vi "Main.vi"() -> ()   [LabVIEW 2018] (continued)
              n599 = Greater Or Equal?(x=w1197, y=w1212) -> (x >= y?=w1196:bool)
              n600 = Divide(x=w1197, y=w1212) -> (x/y=w1209:dbl)
              n601 = Compound Arithmetic op=OR(w1220, "Stop Measure", w1196) -> (w1219:bool)
              n602 = Reshape Array(w1200, w1199, w1199) -> (w1201:dbl[][])
              n603 = Reshape Array(w1202, w1199, w1199) -> (w1203:dbl[][])
              n604 = Reshape Array(w1204, w1199, w1199) -> (w1205:dbl[][])
              n605 = Reshape Array(w1207, w1199, w1199) -> (w1206:dbl[][])
              n606 = Reshape Array(w1218, w1199, w1199) -> (w1208:dbl[][])
              n607 = Multiply(x=w1209, y=100.0) -> (x*y=→"Meas Progress":dbl)
              n608 = local read "V_IF (0.5pi)"() -> (w1214:dbl[][])
              n609 = local read "V_IF (1.5pi)"() -> (w1216:dbl[][])
              n610 = local read "V_IF (pi)"() -> (w1215:dbl[][])
              n611 = local read "V_IF (0)"() -> (w1213:dbl[][])
              n612 = local read "V_DC"() -> (w1217:dbl[][])
              n613 = local read "Shutter Line"() -> (w1177:tag)
              n614 = call "RunningAverage.vi"("New Image"=w1206, "# of Averages for the Old Image"=w1198, "Old Image"=w1216) -> ("Averaged Image"=w1179:dbl[][])  [unwired: 8 in]
              "V_IF (1.5pi)" <- w1179
              n615 = call "RunningAverage.vi"("New Image"=w1201, "# of Averages for the Old Image"=w1198, "Old Image"=w1213) -> ("Averaged Image"=w1182:dbl[][])  [unwired: 8 in]
              "V_IF (0)" <- w1182
              n616 = call "RunningAverage.vi"("New Image"=w1203, "# of Averages for the Old Image"=w1198, "Old Image"=w1214) -> ("Averaged Image"=w1181:dbl[][])  [unwired: 8 in]
              "V_IF (0.5pi)" <- w1181
              n617 = call "RunningAverage.vi"("New Image"=w1205, "# of Averages for the Old Image"=w1198, "Old Image"=w1215) -> ("Averaged Image"=w1180:dbl[][])  [unwired: 8 in]
              "V_IF (pi)" <- w1180
              n618 = call "RunningAverage.vi"("New Image"=w1208, "# of Averages for the Old Image"=w1198, "Old Image"=w1217) -> ("Averaged Image"=w1178:dbl[][])  [unwired: 8 in]
              "V_DC" <- w1178
              n619 = call "ShutterControl.vi"("error in"=w1186, "Shutter Line"=w1177, "Shutter"=FALSE) -> ("error out"=w1188:errorcluster, "Status Indicator"=w1190:bool)  [unwired: 7 in]
              n620 = local write "Shutter"(w1190) -> ()
            }
            n621 = local read "[d13]"() -> (w1141:dbl)
            n622 = local read "[d24]"() -> (w1140:dbl)
            n623 = call "DAQClose.vi"("error in"=w1166, "Functions"=w1167, "Tasks In"=w1168, "DAQ Channels"=w1169) -> ("error out"=w1152:errorcluster)  [unwired: 7 in]
            n624 = local read "[M/B]"() -> (w1145:dbl)
            n625 = local read "[O_B]"() -> (w1144:dbl)
            n626 = call "GSCalculation.vi"("[d24]"=w1140, "[d13]"=w1141, "[O_B]"=w1144, "V_DC"=w1146, "[M/B]"=w1145, "V_IF (1.5pi)"=w1148, "V_IF (pi)"=w1149, "V_IF (0.5pi)"=w1150, "V_IF (0)"=w1151) -> ("S"=w1142:dbl[][], "G"=w1143:dbl[][])  [unwired: 1 in]
            "G Data" <- w1143
            "S Data" <- w1142
          }
          frame #2 {
            n627 = case shown="True" "Calculate Lifetimes and Phasors During Image Acquisition?" {
              tunnel: w1239 -> [w1242 w1272]
              tunnel: w1238 -> [_ w1264]
              tunnel: w1237 -> [_ w1251]
              tunnel: w1236 -> [_ w1250]
              tunnel: w1235 -> [_ w1249]
              tunnel: [w1242 w1244] -> w1234
              frame False {
                # "If need to be fast, e.g., 3D stack acquisition"
              }
              frame True {
                # "If do lifetime and other calcuations"
                n628 = Square(x=w1264) -> (x^2=w1282:i32)
                n629 = call "LifetimeCalculation.vi"("LaserRepRate"="LaserRepRate (Hz)", "S"=w1249, "G"=w1250) -> ("DC&1w Lifetime"=w1273:dbl[][], "1w Lifetime"=w1274:dbl[][])  [unwired: 7 in]
                "1w Lifetime (s)" <- w1274
                "DC&1w Lifetime (s)" <- w1273
                n630 = control-ref of="1w Lifetime Hist"() -> (w1284:refnum<vi>)
                n631 = control-ref of="DC&1w Lifetime Hist"() -> (w1283:refnum<vi>)
                n632 = control-ref of="Lifetime Color Ramp"() -> (w1266:refnum<vi>)
                n633 = control-ref of="Phasor Plot"() -> (w1258:refnum<vi>)
                n634 = local read "Auto Scale?"() -> (w1246:bool)
                n635 = control-ref of="Composite Image"() -> (w1267:refnum<vi>)
                n636 = control-ref of="Image with Phasors"() -> (w1261:refnum<vi>)
                n637 = call "LifetimeHistogram.vi"("1w Lifetime"=w1274, "DC&1w Lifetime"=w1273, "1w reference"=w1284, "DC&1w reference"=w1283, "Max Lifetime (s)"="Max Lifetime (s)", "Min Lifetime (s)"="Min Lifetime (s)", "Data Size"=w1282, "error in (no error)"=w1272, "Bins"="Bins") -> ("error out"=w1268:errorcluster, "1w Lifetime Hist"=→"1w Lifetime Hist":T7, "DC&1w Lifetime Hist"=→"DC&1w Lifetime Hist":T7, "1w mean"=→"u_1w":dbl, "1w std"=→"std_1":dbl, "DC&1w mean"=→"u_01":dbl, "DC&1w std"=→"std_01":dbl)  [unwired: 4 in]
                n638 = case shown="\"1w Lifetime\", Default" "Lifetime Selection" {
                  tunnel: w1274 -> [w1288 _]
                  tunnel: w1273 -> [_ w1289]
                  tunnel: [w1288 w1289] -> w1271
                  frame "1w Lifetime", Default {
                  }
                  frame "DC&1w Lifetime" {
                  }
                }
                n639 = call "HSVCombIntensityLifetime.vi"("min_intensity"="Min Intensity", "Auto Scale?"=w1246, "max_intensity"="Max Intensity", "lifetime_max (s)"="Max Lifetime (s)", "lifetime_min (s)"="Min Lifetime (s)", "Lifetime image"=w1271, "Intensity image"=w1251) -> ("Min"=w1247:dbl, "Max"=w1248:dbl, "Lifetime Color Ramp"=→"Lifetime Color Ramp":i32[][], "HSV to RGB Picture"=→"Composite Image":picture)  [unwired: 1 in]
                n640 = call "Array2GrayPic.vi"("Pic Reference"=w1261, "Threshold (min)"=w1247, "Threshold (max)"=w1248, "Auto Scale?"=w1246, "Intensity"=w1251) -> ("Gray Picture"=→"Image with Phasors":picture)  [unwired: 6 in]
                n641 = local write "Max Intensity"(w1248) -> ()
                n642 = local write "Min Intensity"(w1247) -> ()
                n643 = property on="V_DC" class="IntGraph (strict)"(error in=w1268, "ZScale.Maximum"=w1248, "ZScale.Minimum"=w1247) -> (error out=w1265:errorcluster)  [unwired: 1 in, 1 out]
                n644 = call "CompositeProperties.vi"("Image Reference"=w1267, "Ramp Reference"=w1266, "Pixel Size"=w1264, "Max Lifetime (s)"="Max Lifetime (s)", "Min Lifetime (s)"="Min Lifetime (s)", "error in (no error)"=w1265) -> ("error out"=w1245:errorcluster)  [unwired: 13 in]
                n645 = call "DrawPhasorPlot.vi"("Intensity"=w1251, "G Data"=w1250, "S Data"=w1249, "Threshold (max)"=w1248, "Threshold (min)"=w1247, "error in"=w1245, "G_max"="G_max", "Auto Scale?"=w1246, "G_min"="G_min", "Phasor Grids"="Phasor Grids", "S_max"="S_max", "Reference"=w1258, "S_min"="S_min", "Phasor Colormap"="Phasor Colormap") -> ("Phasor Plot"=→"Phasor Plot":dbl[][], "error out"=w1244:errorcluster)  [unwired: 4 in]
              }
            }
          }
          frame #3 {
            w1297 = FALSE ("Fast Scan")
            n646 = Tick Count (ms)() -> (millisecond timer value=w1293:u32)
            n647 = local write "Measure"(w1297) -> ()
            n648 = local write "Stop Measure"(w1297) -> ()
            n649 = Subtract(x=w1293, y=w1292) -> (x-y=w1294:u32)
            n650 = To Double Precision Float(number=w1294) -> (double precision float=w1295:dbl)
            n651 = Divide(x=w1295, y=1000.0) -> (x/y=→"Actual Meas Time (s)":dbl)
          }
        }
      }
      event "Refresh": Value Change {
        n652 = event-data() -> ()  [unwired: 1 in, 1 out]
        n653 = flat-sequence {
          tunnel: [w1348] -> w1306
          tunnel: w1305 -> [w1348]
          tunnel: [w1346] -> w1303
          tunnel: w1302 -> [w1347]
          tunnel: w1306 -> [w1359]
          tunnel: [w1359] -> w1304
          tunnel: w1303 -> [w1358]
          tunnel: [w1358] -> w1301
          frame #0 {
            n654 = local read "Measurement Parameters"() -> (w1350:T4)
            n655 = local read "LaserRepRate (Hz)"() -> (w1307:dbl)
            n656 = Unbundle By Name(w1350) -> ("Pixel Size"=w1349:dbl)
            n657 = local read "G Data"() -> (w1352:dbl[][])
            n658 = local read "V_DC"() -> (w1354:dbl[][])
            n659 = local read "S Data"() -> (w1353:dbl[][])
            n660 = To Long Integer(number=w1349) -> (32bit integer=w1351:i32)
            n661 = Square(x=w1351) -> (x^2=w1345:i32)
            n662 = local read "Phasor Colormap"() -> (w1310:T8)
            n663 = local read "Max Lifetime (s)"() -> (w1339:dbl)
            n664 = local read "Min Lifetime (s)"() -> (w1338:dbl)
            n665 = control-ref of="Phasor Plot"() -> (w1309:refnum<vi>)
            n666 = control-ref of="Lifetime Color Ramp"() -> (w1319:refnum<vi>)
            n667 = call "LifetimeCalculation.vi"("LaserRepRate"=w1307, "S"=w1353, "G"=w1352) -> ("DC&1w Lifetime"=w1334:dbl[][], "1w Lifetime"=w1335:dbl[][])  [unwired: 7 in]
            n668 = local read "Bins"() -> (w1333:i32)
            n669 = control-ref of="1w Lifetime Hist"() -> (w1326:refnum<vi>)
            n670 = control-ref of="DC&1w Lifetime Hist"() -> (w1325:refnum<vi>)
            n671 = local read "Phasor Grids"() -> (w1311:i32)
            n672 = local read "Max Intensity"() -> (w1337:dbl)
            n673 = local read "Min Intensity"() -> (w1336:dbl)
            n674 = local read "Auto Scale?"() -> (w1341:bool)
            n675 = local read "G_max"() -> (w1315:dbl)
            n676 = local read "S_max"() -> (w1313:dbl)
            n677 = local read "G_min"() -> (w1314:dbl)
            n678 = local read "S_min"() -> (w1312:dbl)
            n679 = control-ref of="Image with Phasors"() -> (w1318:refnum<vi>)
            n680 = control-ref of="Composite Image"() -> (w1320:refnum<vi>)
            n681 = call "LifetimeHistogram.vi"("1w Lifetime"=w1335, "DC&1w Lifetime"=w1334, "1w reference"=w1326, "DC&1w reference"=w1325, "Max Lifetime (s)"=w1339, "Min Lifetime (s)"=w1338, "Data Size"=w1345, "error in (no error)"=w1347, "Bins"=w1333) -> ("error out"=w1343:errorcluster, "1w Lifetime Hist"=w1332:T7, "DC&1w Lifetime Hist"=w1331:T7, "1w mean"=w1330:dbl, "1w std"=w1329:dbl, "DC&1w mean"=w1328:dbl, "DC&1w std"=w1327:dbl)  [unwired: 4 in]
            n682 = local write "1w Lifetime (s)"(w1335) -> ()
            n683 = local write "DC&1w Lifetime (s)"(w1334) -> ()
            n684 = local write "1w Lifetime Hist"(w1332) -> ()
            n685 = local write "DC&1w Lifetime Hist"(w1331) -> ()
            n686 = local write "u_1w"(w1330) -> ()
            n687 = local write "std_1"(w1329) -> ()
            n688 = local write "u_01"(w1328) -> ()
            n689 = local write "std_01"(w1327) -> ()
            n690 = local read "Lifetime Selection"() -> (w1308:enum32{"1w Lifetime", "DC&1w Lifetime"})
            n691 = case shown="\"1w Lifetime\", Default" w1308 {
              tunnel: w1335 -> [w1355 _]
              tunnel: w1334 -> [_ w1356]
              tunnel: [w1355 w1356] -> w1344
              frame "1w Lifetime", Default {
              }
              frame "DC&1w Lifetime" {
              }
            }
            n692 = call "HSVCombIntensityLifetime.vi"("min_intensity"=w1336, "Auto Scale?"=w1341, "max_intensity"=w1337, "lifetime_max (s)"=w1339, "lifetime_min (s)"=w1338, "Lifetime image"=w1344, "Intensity image"=w1354) -> ("Min"=w1321:dbl, "Max"=w1322:dbl, "Lifetime Color Ramp"=w1323:i32[][], "HSV to RGB Picture"=w1324:picture)  [unwired: 1 in]
            n693 = call "Array2GrayPic.vi"("Pic Reference"=w1318, "Threshold (min)"=w1321, "Threshold (max)"=w1322, "Auto Scale?"=w1341, "Intensity"=w1354) -> ("Gray Picture"=w1317:picture)  [unwired: 6 in]
            n694 = local write "Image with Phasors"(w1317) -> ()
            n695 = property on="V_DC" class="IntGraph (strict)"(error in=w1343, "ZScale.Maximum"=w1322, "ZScale.Minimum"=w1321) -> (error out=w1342:errorcluster)  [unwired: 1 in, 1 out]
            n696 = call "CompositeProperties.vi"("Image Reference"=w1320, "Ramp Reference"=w1319, "Pixel Size"=w1351, "Max Lifetime (s)"=w1339, "Min Lifetime (s)"=w1338, "error in (no error)"=w1342) -> ("error out"=w1340:errorcluster)  [unwired: 13 in]
            n697 = call "DrawPhasorPlot.vi"("Intensity"=w1354, "G Data"=w1352, "S Data"=w1353, "Threshold (max)"=w1322, "Threshold (min)"=w1321, "error in"=w1340, "G_max"=w1315, "Auto Scale?"=w1341, "G_min"=w1314, "Phasor Grids"=w1311, "S_max"=w1313, "Reference"=w1309, "S_min"=w1312, "Phasor Colormap"=w1310) -> ("Phasor Plot"=w1316:dbl[][], "error out"=w1346:errorcluster)  [unwired: 4 in]
            n698 = local write "Phasor Plot"(w1316) -> ()
            n699 = local write "Composite Image"(w1324) -> ()
            n700 = local write "Lifetime Color Ramp"(w1323) -> ()
            n701 = local write "Max Intensity"(w1322) -> ()
            n702 = local write "Min Intensity"(w1321) -> ()
          }
          frame #1 {
            n703 = local write "Refresh"(FALSE ("Fast Scan")) -> ()
          }
        }
      }
      event "Z-Stack Measure": Value Change {
        n704 = event-data() -> ()  [unwired: 1 in, 1 out]
        n705 = local read "Current Slice"() -> (w1370:i32)
        n706 = Divide(x=w1370, y="Z Slice Number") -> (x/y=w1378:dbl)
        n707 = Greater Or Equal?(x=w1370, y="Z Slice Number") -> (x >= y?=w1371:bool)
        n708 = Multiply(x=w1378, y=100.0) -> (x*y=→"Stack Progress":dbl)
        n709 = local read "Use Stage?"() -> (w1360:bool)
        n710 = Equal To 0?(x=w1370) -> (x = 0?=w1369:bool)
        n711 = case shown="True" w1369 {
          tunnel: w1380 -> [w1440 w1473]
          tunnel: w1381 -> [w1439 w1474]
          tunnel: [w1438 w1472] -> w1374
          tunnel: [w1437 w1471] -> w1372
          tunnel: w1371 -> [w1433 _]
          tunnel: [FALSE ("Stop Stack Measure") w1468] -> w1362
          tunnel: w1360 -> [w1425 w1466]
          frame False {
            # "Continue measurement , move stage"
            n712 = case shown="False" w1433 {
              tunnel: w1440 -> [w1445 w1464]
              tunnel: w1439 -> [w1444 w1465]
              tunnel: [w1443 w1465] -> w1438
              tunnel: [w1442 w1464] -> w1437
              tunnel: w1425 -> [w1441 _]
              frame False {
                n713 = case shown="True" w1441 {
                  tunnel: w1445 -> [w1446 w1463]
                  tunnel: w1444 -> [w1447 w1462]
                  tunnel: [w1447 w1450] -> w1443
                  tunnel: [w1446 w1448] -> w1442
                  frame False {
                  }
                  frame True {
                    # "Moves up by 1 step defined by \nthe 'C' command"
                    n714 = Number To Decimal String(number="Z Slice Size (.1um)") -> (decimal integer string=w1456:string)  [unwired: 1 in]
                    n715 = Concatenate Strings("C" ("string"), "," ("string"), w1456, "\r", "U" ("string")) -> (w1453:string)
                    n716 = VISA Write(VISA resource name=w1462, write buffer=w1453, error in (no error)=w1463) -> (VISA resource name out=w1460:refnum<visa-resource-name>, error out=w1459:errorcluster)  [unwired: 1 out]
                    n717 = VISA Read(VISA resource name=w1460, byte count=u32 256, error in (no error)=w1459) -> (VISA resource name out=w1451:refnum<visa-resource-name>, error out=w1449:errorcluster)  [unwired: 2 out]
                    n718 = VISA Clear(VISA resource name=w1451, error in (no error)=w1449) -> (VISA resource name out=w1450:refnum<visa-resource-name>, error out=w1448:errorcluster)
                  }
                }
              }
              frame True {
              }
            }
            n719 = local read "3D Intensity"() -> (w1434:dbl[][][])
            n720 = local read "G Data"() -> (w1432:dbl[][])
            n721 = local read "S Data"() -> (w1431:dbl[][])
            n722 = local read "V_DC"() -> (w1436:dbl[][])
            n723 = local read "3D G"() -> (w1428:dbl[][][])
            n724 = local read "3D S"() -> (w1427:dbl[][][])
            n725 = Build Array (concatenate)(w1434, w1436) -> (→"3D Intensity":dbl[][][])
            n726 = Build Array (concatenate)(w1428, w1432) -> (→"3D G":dbl[][][])
            n727 = Build Array (concatenate)(w1427, w1431) -> (→"3D S":dbl[][][])
          }
          frame True {
            # "Beginning the measurment, record current Z position"
            n728 = local read "3D Time-Lapse Measure"() -> (w1467:bool)
            n729 = case shown="False" w1467 {
              tunnel: [w1487 TRUE ("T button?")] -> w1469
              frame False {
                n730 = Two Button Dialog(message="Discard Previous Stack?") -> (T button?=w1487:bool)  [unwired: 2 in]
              }
              frame True {
              }
            }
            n731 = case shown="True" w1466 {
              tunnel: w1474 -> [w1476 w1482]
              tunnel: w1473 -> [w1475 w1481]
              tunnel: [w1476 w1480] -> w1472
              tunnel: [w1475 w1479] -> w1471
              frame False {
              }
              frame True {
                n732 = VISA Write(VISA resource name=w1482, write buffer="PZ" ("string"), error in (no error)=w1481) -> (VISA resource name out=w1484:refnum<visa-resource-name>, error out=w1485:errorcluster)  [unwired: 1 out]
                n733 = VISA Read(VISA resource name=w1484, byte count=u32 256, error in (no error)=w1485) -> (VISA resource name out=w1480:refnum<visa-resource-name>, read buffer=w1478:string, error out=w1479:errorcluster)  [unwired: 1 out]
                n734 = Decimal String To Number(string=w1478) -> (number=→"Initial Z Pos (.1um)":i32)  [unwired: 2 in, 1 out]
              }
            }
            n735 = local write "Calculate Lifetimes and Phasors During Image Acquisition?"(FALSE ("Calculate Lifetimes and Phasors During Image Acquisition?")) -> ()
            n736 = case shown="True" w1469 {
              tunnel: [TRUE ("Stop Stack Measure") FALSE ("Stop Stack Measure")] -> w1468
              frame False {
              }
              frame True {
                w1492 = dbl[][][] [] ("3D Intensity (BT)")
                n737 = local write "3D Intensity"(w1492) -> ()
                n738 = local write "3D G"(w1492) -> ()
                n739 = local write "3D S"(w1492) -> ()
              }
            }
          }
        }
        n740 = Compound Arithmetic op=OR(w1371, "Stop Stack Measure", w1362) -> (w1375:bool)
        n741 = case shown="True" w1375 {
          tunnel: w1374 -> [w1394 w1399]
          tunnel: w1372 -> [w1389 w1398]
          tunnel: [w1394 w1404] -> w1368
          tunnel: [w1391 w1400] -> w1366
          tunnel: w1370 -> [w1393 _]
          frame False {
            n742 = Increment(x=w1393) -> (x+1=→"Current Slice":i32)
            n743 = property on="Measure" class="Bool (strict)"(error in=w1389, "Val(Sgnl)"=TRUE ("Value (Signaling)")) -> (error out=w1388:errorcluster)  [unwired: 1 in, 1 out]
            n744 = property on="Z-Stack Measure" class="Bool (strict)"(error in=w1388, "Val(Sgnl)"=TRUE ("Value (Signaling)")) -> (error out=w1391:errorcluster)  [unwired: 1 in, 1 out]
          }
          frame True {
            w1403 = FALSE ("Fast Scan")
            n745 = local read "Use Stage?"() -> (w1396:bool)
            n746 = case shown="True" w1396 {
              tunnel: [w1407 w1411] -> w1404
              tunnel: [w1406 w1410] -> w1401
              tunnel: w1399 -> [w1407 w1409]
              tunnel: w1398 -> [w1406 w1408]
              frame False {
              }
              frame True {
                n747 = local read "Initial Z Pos (.1um)"() -> (w1419:i32)
                n748 = Number To Decimal String(number=w1419) -> (decimal integer string=w1416:string)  [unwired: 1 in]
                n749 = Concatenate Strings("GZ" ("string"), "," ("string"), w1416) -> (w1418:string)
                n750 = VISA Write(VISA resource name=w1409, write buffer=w1418, error in (no error)=w1408) -> (VISA resource name out=w1413:refnum<visa-resource-name>, error out=w1414:errorcluster)  [unwired: 1 out]
                n751 = VISA Read(VISA resource name=w1413, byte count=u32 256, error in (no error)=w1414) -> (VISA resource name out=w1411:refnum<visa-resource-name>, error out=w1410:errorcluster)  [unwired: 2 out]
              }
            }
            n752 = local read "3D Time-Lapse Measure"() -> (w1402:bool)
            n753 = local write "Calculate Lifetimes and Phasors During Image Acquisition?"(TRUE ("Calculate Lifetimes and Phasors During Image Acquisition?")) -> ()
            n754 = local write "Stop Stack Measure"(w1403) -> ()
            n755 = local write "Z-Stack Measure"(w1403) -> ()
            n756 = local write "Current Slice"(0 ("Current Slice")) -> ()
            n757 = case shown="True" w1402 {
              tunnel: w1401 -> [w1420 w1422]
              tunnel: [w1420 w1421] -> w1400
              frame False {
              }
              frame True {
                w1423 = TRUE ("Value (Signaling)")
                n758 = property on="Save 3D Stacks" class="Bool (strict)"(error in=w1422, "Val(Sgnl)"=w1423) -> (error out=w1424:errorcluster)  [unwired: 1 in, 1 out]
                n759 = property on="3D Time-Lapse Measure" class="Bool (strict)"(error in=w1424, "Val(Sgnl)"=w1423) -> (error out=w1421:errorcluster)  [unwired: 1 in, 1 out]
              }
            }
          }
        }
        n760 = local read "Use Stage?"() -> (w1361:bool)
        n761 = case shown="False" w1361 {
          tunnel: w1368 -> [w1382 w1387]
          tunnel: [w1382 w1386] -> w1367
          tunnel: w1366 -> [w1383 w1385]
          tunnel: [w1383 w1384] -> w1365
          frame False {
          }
          frame True {
            n762 = VISA Clear(VISA resource name=w1387, error in (no error)=w1385) -> (VISA resource name out=w1386:refnum<visa-resource-name>, error out=w1384:errorcluster)
          }
        }
      }
      event "3D Stack to Show", "Slice Slider": Value Change {
        n763 = event-data() -> ()  [unwired: 1 in, 1 out]
        n764 = local read "3D Intensity"() -> (w1515:dbl[][][])
        n765 = local read "Max Lifetime (s)"() -> (w1517:dbl)
        n766 = local read "Min Lifetime (s)"() -> (w1516:dbl)
        n767 = local read "LaserRepRate (Hz)"() -> (w1493:dbl)
        n768 = case shown="False" "Auto Scale?" {
          tunnel: w1515 -> [_ w1535]
          tunnel: [w1532 w1534] -> w1514
          tunnel: [w1531 w1533] -> w1513
          frame False {
            n769 = local read "Max Intensity"() -> (w1532:dbl)
            n770 = local read "Min Intensity"() -> (w1531:dbl)
          }
          frame True {
            n771 = Array Max & Min(array=w1535) -> (max value=w1534:dbl, min value=w1533:dbl)  [unwired: 2 out]
          }
        }
        n772 = local read "3D G"() -> (w1499:dbl[][][])
        n773 = local read "3D S"() -> (w1498:dbl[][][])
        n774 = control-ref of="Slice of 3D Stack"() -> (w1500:refnum<vi>)
        n775 = Multiply(x=w1493, y=6.283185307179586) -> (x*y=w1496:dbl)
        n776 = case shown="\"Overlap 3D\"" "3D Stack to Show" {
          tunnel: "Slice Slider" -> [w1545 w1558 w1574 w1591 w1612 w1632 w1651]
          tunnel: [w1543 w1557 w1573 w1592 w1611 w1635 w1654] -> w1518
          tunnel: w1517 -> [_ w1553 w1570 w1584 w1602 _ _]
          tunnel: w1516 -> [_ w1552 w1569 w1583 w1595 _ _]
          tunnel: w1515 -> [w1542 _ _ w1590 w1610 w1636 w1655]
          tunnel: w1514 -> [w1538 _ _ w1587 w1605 w1621 w1646]
          tunnel: w1513 -> [w1537 _ _ w1586 w1604 w1620 w1645]
          tunnel: [w1536 w1551 w1568 w1581 w1607 w1616 w1648] -> w1502
          tunnel: w1500 -> [w1540 w1555 w1567 w1589 w1608 w1617 w1650]
          tunnel: w1499 -> [_ w1549 w1564 w1579 w1597 w1634 w1653]
          tunnel: w1498 -> [_ w1548 _ w1578 _ w1633 w1652]
          tunnel: w1496 -> [_ w1547 w1561 w1577 w1596 _ _]
          frame "Intensity 3D", Default {
            n777 = Array Size(array=w1542) -> (size(s)=w1544:i32[])
            n778 = Index Array(array=w1542, index (dim 0)=w1545) -> (element=w1541:dbl[][])  [unwired: 2 in]
            n779 = Index Array(array=w1544) -> (element=w1543:i32)  [unwired: 1 in]
            n780 = call "Array2GrayPic.vi"("Pic Reference"=w1540, "Threshold (min)"=w1537, "Threshold (max)"=w1538, "Auto Scale?"=FALSE, "Intensity"=w1541) -> ("Gray Picture"=w1536:picture)  [unwired: 6 in]
          }
          frame "1w Lifetime 3D" {
            n781 = Divide(x=w1548, y=w1549) -> (x/y=w1550:dbl[][][])
            n782 = Divide(x=w1550, y=w1547) -> (x/y=w1546:dbl[][][])
            n783 = Array Size(array=w1546) -> (size(s)=w1559:i32[])
            n784 = Index Array(array=w1546, index (dim 0)=w1558) -> (element=w1554:dbl[][])  [unwired: 2 in]
            n785 = Index Array(array=w1559) -> (element=w1557:i32)  [unwired: 1 in]
            n786 = call "Array2GrayPic.vi"("Pic Reference"=w1555, "Threshold (min)"=w1552, "Threshold (max)"=w1553, "Auto Scale?"=FALSE, "Intensity"=w1554) -> ("Gray Picture"=w1551:picture)  [unwired: 6 in]
          }
          frame "DC&1w Lifetime 3D" {
            n787 = Divide(x=1.0, y=w1564) -> (x/y=w1563:dbl[][][])
            n788 = Decrement(x=w1563) -> (x-1=w1566:dbl[][][])
            n789 = Square Root(x=w1566) -> (sqrt(x)=w1562:dbl[][][])
            n790 = Divide(x=w1562, y=w1561) -> (x/y=w1560:dbl[][][])
            n791 = Array Size(array=w1560) -> (size(s)=w1575:i32[])
            n792 = Index Array(array=w1560, index (dim 0)=w1574) -> (element=w1571:dbl[][])  [unwired: 2 in]
            n793 = Index Array(array=w1575) -> (element=w1573:i32)  [unwired: 1 in]
            n794 = call "Array2GrayPic.vi"("Pic Reference"=w1567, "Threshold (min)"=w1569, "Threshold (max)"=w1570, "Auto Scale?"=FALSE, "Intensity"=w1571) -> ("Gray Picture"=w1568:picture)  [unwired: 6 in]
          }
          frame "1w Composite 3D" {
            n795 = Divide(x=w1578, y=w1579) -> (x/y=w1580:dbl[][][])
            n796 = Divide(x=w1580, y=w1577) -> (x/y=w1576:dbl[][][])
            n797 = Index Array(array=w1576, index (dim 0)=w1591) -> (element=w1585:dbl[][])  [unwired: 2 in]
            n798 = Index Array(array=w1590, index (dim 0)=w1591) -> (element=w1588:dbl[][])  [unwired: 2 in]
            n799 = Array Size(array=w1590) -> (size(s)=w1593:i32[])
            n800 = Index Array(array=w1593) -> (element=w1592:i32)  [unwired: 1 in]
            n801 = call "Array2HSVColorPic.vi"("Intensity"=w1588, "Threshold (max)"=w1587, "Threshold (min)"=w1586, "Lifetime"=w1585, "lifetime_max (s)"=w1584, "lifetime_min (s)"=w1583, "Pic Reference"=w1589, "Auto Scale?"=FALSE) -> ("Gray Picture"=w1581:picture)  [unwired: 11 in]
          }
          frame "DC&1w Composite 3D" {
            n802 = Divide(x=1.0, y=w1597) -> (x/y=w1599:dbl[][][])
            n803 = Decrement(x=w1599) -> (x-1=w1601:dbl[][][])
            n804 = Square Root(x=w1601) -> (sqrt(x)=w1598:dbl[][][])
            n805 = Divide(x=w1598, y=w1596) -> (x/y=w1594:dbl[][][])
            n806 = Index Array(array=w1594, index (dim 0)=w1612) -> (element=w1603:dbl[][])  [unwired: 2 in]
            n807 = Index Array(array=w1610, index (dim 0)=w1612) -> (element=w1606:dbl[][])  [unwired: 2 in]
            n808 = Array Size(array=w1610) -> (size(s)=w1613:i32[])
            n809 = Index Array(array=w1613) -> (element=w1611:i32)  [unwired: 1 in]
            n810 = call "Array2HSVColorPic.vi"("Intensity"=w1606, "Threshold (max)"=w1605, "Threshold (min)"=w1604, "Lifetime"=w1603, "lifetime_max (s)"=w1602, "lifetime_min (s)"=w1595, "Pic Reference"=w1608, "Auto Scale?"=FALSE) -> ("Gray Picture"=w1607:picture)  [unwired: 11 in]
          }
          frame "Phasor 3D" {
            # "Transpose"
            n811 = Array Size(array=w1636) -> (size(s)=w1637:i32[])
            n812 = Index Array(array=w1633, index (dim 0)=w1632) -> (element=w1622:dbl[][])  [unwired: 2 in]
            n813 = Index Array(array=w1634, index (dim 0)=w1632) -> (element=w1623:dbl[][])  [unwired: 2 in]
            n814 = Index Array(array=w1636, index (dim 0)=w1632) -> (element=w1624:dbl[][])  [unwired: 2 in]
            n815 = Index Array(array=w1637) -> (element=w1635:i32)  [unwired: 1 in]
            n816 = local read "Phasor Colormap"() -> (w1625:T8)
            n817 = local read "G_max"() -> (w1631:dbl)
            n818 = local read "S_max"() -> (w1629:dbl)
            n819 = local read "G_min"() -> (w1630:dbl)
            n820 = local read "S_min"() -> (w1628:dbl)
            n821 = control-ref of="Phasor Plot"() -> (w1626:refnum<vi>)
            n822 = local read "Phasor Grids"() -> (w1627:i32)
            n823 = call "DrawPhasorPlot.vi"("Intensity"=w1624, "G Data"=w1623, "S Data"=w1622, "Threshold (max)"=w1621, "Threshold (min)"=w1620, "G_max"=w1631, "Auto Scale?"=FALSE, "G_min"=w1630, "Phasor Grids"=w1627, "S_max"=w1629, "Reference"=w1626, "S_min"=w1628, "Phasor Colormap"=w1625) -> ("Phasor Plot"=w1614:dbl[][])  [unwired: 5 in, 1 out]
            n824 = Transpose 2D Array(2D array=w1614) -> (transposed array=w1615:dbl[][])
            n825 = call "Array2GrayPic.vi"("Pic Reference"=w1617, "Auto Scale?"=TRUE, "Intensity"=w1615) -> ("Gray Picture"=w1616:picture)  [unwired: 8 in]
          }
          frame "Overlap 3D" {
            n826 = Array Size(array=w1655) -> (size(s)=w1656:i32[])
            n827 = Index Array(array=w1655, index (dim 0)=w1651) -> (element=w1649:dbl[][])  [unwired: 2 in]
            n828 = Index Array(array=w1652, index (dim 0)=w1651) -> (element=w1643:dbl[][])  [unwired: 2 in]
            n829 = Index Array(array=w1653, index (dim 0)=w1651) -> (element=w1644:dbl[][])  [unwired: 2 in]
            n830 = Index Array(array=w1656) -> (element=w1654:i32)  [unwired: 1 in]
            n831 = local read "ROI Cluster"() -> (w1642:T9)
            n832 = Unbundle(w1642) -> (w1641:bool[], w1640:dbl[], w1639:cluster{dbl, dbl}[], w1638:u32[])
            n833 = call "PhasorROI2IMG.vi"("Intensity"=w1649, "Auto Scale?"=FALSE, "Threshold (max)"=w1646, "Threshold (min)"=w1645, "G Data"=w1644, "S Data"=w1643, "Pic Reference"=w1650, "ROI? array"=w1641, "Radius array"=w1640, "Center array"=w1639, "Color array"=w1638) -> ("new picture"=w1648:picture)  [unwired: 8 in]
          }
        }
        "Slice of 3D Stack" <- w1502
        "Number of Slices" <- w1518
        n834 = local read "Measurement Parameters"() -> (w1512:T4)
        n835 = property on="Slice of 3D Stack" class="Pict"(error in=w1506) -> (error out=w1505:errorcluster, "Draw Area Size"=w1510:T16)  [unwired: 1 in, 1 out]
        n836 = Unbundle By Name(w1510) -> ("Width"=w1507:u32)
        n837 = Unbundle By Name(w1512) -> ("Pixel Size"=w1503:dbl)
        n838 = To Single Precision Float(number=w1507) -> (single precision float=w1509:sgl)
        n839 = To Single Precision Float(number=w1503) -> (single precision float=w1508:sgl)
        n840 = Divide(x=w1509, y=w1508) -> (x/y=w1511:sgl)
        n841 = property on="Slice of 3D Stack" class="Pict"(error in=w1505, "ZoomFactor"=w1511) -> (error out=w1504:errorcluster)  [unwired: 1 in, 1 out]
        n842 = Increment(x="Slice Slider") -> (x+1=w1524:i32)
        n843 = Number To Decimal String(number=w1524) -> (decimal integer string=w1522:string)  [unwired: 1 in]
        n844 = Number To Decimal String(number=w1518) -> (decimal integer string=w1527:string)  [unwired: 1 in]
        n845 = property on="Slice Slider" class="Scroll (strict)"(error in=w1504, "DocMax"=w1518) -> (error out=w1521:errorcluster)  [unwired: 1 in, 1 out]
        n846 = Concatenate Strings("Slice #: " ("string"), w1522, "/" ("string"), w1527) -> (→"Slice Display":string)
        n847 = property on="Slice Slider" class="Scroll (strict)"(error in=w1521, "DocMin"=0.0 ("Doc Min")) -> (error out=w1520:errorcluster)  [unwired: 1 in, 1 out]
      }
      event "Save 3D Stacks": Value Change {
        # "Always save raw data for 3D"
        n848 = event-data() -> ()  [unwired: 1 in, 1 out]
        n849 = local read "3D Intensity"() -> (w1685:dbl[][][])
        n850 = local read "Current 3D Time-Lapse Meas"() -> (w1687:i32)
        n851 = local read "Crop Pixels"() -> (w1672:u16)
        n852 = local read "3D G"() -> (w1677:dbl[][][])
        n853 = local read "3D S"() -> (w1675:dbl[][][])
        n854 = case shown="True" TRUE {
          tunnel: [w1691 w1693] -> w1684
          tunnel: [w1690 w1692] -> w1683
          tunnel: w1685 -> [_ w1694]
          frame False {
            n855 = local read "Max Intensity"() -> (w1691:dbl)
            n856 = local read "Min Intensity"() -> (w1690:dbl)
          }
          frame True {
            n857 = Array Max & Min(array=w1694) -> (max value=w1693:dbl, min value=w1692:dbl)  [unwired: 2 out]
          }
        }
        n858 = case shown="True" "Current Directory (3D)?" {
          tunnel: ["Save Directory (3D)" w1696] -> w1673
          frame False {
          }
          frame True {
            n859 = Current VI's Path() -> (path=w1697:path)
            n860 = Strip Path(path=w1697) -> (stripped path=w1696:path)  [unwired: 1 out]
          }
        }
        n861 = Number To Decimal String(number=w1687) -> (decimal integer string=w1670:string)  [unwired: 1 in]
        n862 = call "Save3DStack.vi"("Experiment Name"="Experiment Name (3D)", "Identify Name"="I" ("string"), "3D Data"=w1685, "matrix_max"=w1684, "matrix_min"=w1683, "error in"=w1682, "File Name"="File Name (3D)", "Index Name"=w1670, "path"=w1673, "Specify Range?"=TRUE ("Bound Pixel Value?"), "Enable?"=TRUE, "Crop Pixels"=w1672, "Time Stamp?"=FALSE ("Enable?")) -> ("error out"=w1678:errorcluster)  [unwired: 5 in, 1 out]
        n863 = call "Save3DStack.vi"("Experiment Name"="Experiment Name (3D)", "Identify Name"="G" ("string"), "3D Data"=w1677, "error in"=w1678, "File Name"="File Name (3D)", "Index Name"=w1670, "path"=w1673, "Specify Range?"=FALSE ("Bound Pixel Value?"), "Enable?"=TRUE, "Crop Pixels"=w1672, "Time Stamp?"=FALSE ("Enable?")) -> ("error out"=w1665:errorcluster)  [unwired: 7 in, 1 out]
        n864 = call "Save3DStack.vi"("Experiment Name"="Experiment Name (3D)", "Identify Name"="S" ("string"), "3D Data"=w1675, "error in"=w1665, "File Name"="File Name (3D)", "Index Name"=w1670, "path"=w1673, "Specify Range?"=FALSE ("Bound Pixel Value?"), "Enable?"=TRUE, "Crop Pixels"=w1672, "Time Stamp?"=FALSE ("Enable?")) -> ("error out"=w1676:errorcluster)  [unwired: 7 in, 1 out]
        n865 = flat-sequence {
          tunnel: w1676 -> [w1699]
          tunnel: [w1699] -> w1660
          frame #0 {
            n866 = local write "Save 3D Stacks"(FALSE ("Save 3D Stacks")) -> ()
          }
        }
      }
      event "2D Time-Lapse Measure": Value Change {
        n867 = event-data() -> ()  [unwired: 1 in, 1 out]
        n868 = local read "Current 2D Time-Lapse Meas"() -> (w1705:i32)
        n869 = Divide(x=w1705, y="Total 2D Time-Lapse Meas") -> (x/y=w1710:dbl)
        n870 = Greater Or Equal?(x=w1705, y="Total 2D Time-Lapse Meas") -> (x >= y?=w1711:bool)
        n871 = Multiply(x=w1710, y=100.0) -> (x*y=→"2D Time-Lapse Progress":dbl)
        n872 = Compound Arithmetic op=OR(w1711, "Stop 2D Time-Lapse") -> (w1707:bool)
        n873 = case shown="False" w1707 {
          tunnel: w1705 -> [w1716 _]
          tunnel: w1703 -> [w1717 w1736]
          tunnel: [w1718 w1736] -> w1702
          frame False {
            w1719 = TRUE ("Value (Signaling)")
            n874 = Equal To 0?(x=w1716) -> (x = 0?=w1715:bool)
            n875 = case shown="False" w1715 {
              tunnel: [w1726 w1735] -> w1714
              tunnel: w1717 -> [w1726 w1735]
              frame False {
                n876 = while {
                  stop <- w1728 stop-if-true
                  n877 = local read "Time Stamp (s)"() -> (w1732:dbl)
                  n878 = Get Date/Time In Seconds() -> (seconds since 1Jan1904=w1734:timestamp)
                  n879 = local read "Stop 2D Time-Lapse"() -> (w1727:bool)
                  n880 = To Double Precision Float(number=w1734) -> (double precision float=w1733:dbl)
                  n881 = Subtract(x=w1733, y=w1732) -> (x-y=w1731:dbl)
                  "Time Elapse (s)" <- w1731
                  n882 = Greater Or Equal?(x=w1731, y="2D Time-Lapse Interval (s)") -> (x >= y?=w1729:bool)
                  n883 = Compound Arithmetic op=OR(w1729, w1727) -> (w1728:bool)
                }
              }
              frame True {
              }
            }
            n884 = Increment(x=w1716) -> (x+1=→"Current 2D Time-Lapse Meas":i32)
            n885 = flat-sequence {
              tunnel: [w1725] -> w1713
              tunnel: w1714 -> [w1725]
              frame #0 {
                n886 = Get Date/Time In Seconds() -> (seconds since 1Jan1904=w1723:timestamp)
                n887 = To Double Precision Float(number=w1723) -> (double precision float=→"Time Stamp (s)":dbl)
              }
            }
            n888 = property on="Measure" class="Bool (strict)"(error in=w1713, "Val(Sgnl)"=w1719) -> (error out=w1721:errorcluster)  [unwired: 1 in, 1 out]
            n889 = property on="Save 2D Images" class="Bool (strict)"(error in=w1721, "Val(Sgnl)"=w1719) -> (error out=w1720:errorcluster)  [unwired: 1 in, 1 out]
            n890 = property on="2D Time-Lapse Measure" class="Bool (strict)"(error in=w1720, "Val(Sgnl)"=w1719) -> (error out=w1718:errorcluster)  [unwired: 1 in, 1 out]
          }
          frame True {
            w1737 = FALSE ("2D Time-Lapse Measure")
            n891 = local write "Current 2D Time-Lapse Meas"(0 ("Current Slice")) -> ()
            n892 = local write "2D Time-Lapse Measure"(w1737) -> ()
            n893 = local write "Stop 2D Time-Lapse"(w1737) -> ()
          }
        }
      }
      event "3D Time-Lapse Measure": Value Change {
        n894 = event-data() -> ()  [unwired: 1 in, 1 out]
        n895 = local read "Current 3D Time-Lapse Meas"() -> (w1749:i32)
        n896 = Divide(x=w1749, y="Total 3D Time-Lapse Meas") -> (x/y=w1743:dbl)
        n897 = Greater Or Equal?(x=w1749, y="Total 3D Time-Lapse Meas") -> (x >= y?=w1747:bool)
        n898 = Multiply(x=w1743, y=100.0) -> (x*y=→"3D Time-Lapse Progress":dbl)
        n899 = Compound Arithmetic op=OR(w1747, "Stop 3D Time-Lapse") -> (w1750:bool)
        n900 = case shown="False" w1750 {
          tunnel: w1749 -> [w1758 _]
          tunnel: w1742 -> [w1755 w1773]
          tunnel: [w1752 w1773] -> w1741
          frame False {
            n901 = Equal To 0?(x=w1758) -> (x = 0?=w1757:bool)
            n902 = case shown="False" w1757 {
              tunnel: w1755 -> [w1763 w1772]
              tunnel: [w1763 w1772] -> w1754
              frame False {
                n903 = while {
                  stop <- w1764 stop-if-true
                  n904 = local read "Time Stamp (s)"() -> (w1769:dbl)
                  n905 = Get Date/Time In Seconds() -> (seconds since 1Jan1904=w1771:timestamp)
                  n906 = local read "Stop 3D Time-Lapse"() -> (w1765:bool)
                  n907 = To Double Precision Float(number=w1771) -> (double precision float=w1770:dbl)
                  n908 = Subtract(x=w1770, y=w1769) -> (x-y=w1767:dbl)
                  n909 = Greater Or Equal?(x=w1767, y="3D Time-Lapse Interval (s)") -> (x >= y?=w1768:bool)
                  n910 = local write "Time Elapse (s)"(w1767) -> ()
                  n911 = Compound Arithmetic op=OR(w1768, w1765) -> (w1764:bool)
                }
              }
              frame True {
              }
            }
            n912 = Increment(x=w1758) -> (x+1=→"Current 3D Time-Lapse Meas":i32)
            n913 = flat-sequence {
              tunnel: [w1760] -> w1753
              tunnel: w1754 -> [w1760]
              frame #0 {
                n914 = Get Date/Time In Seconds() -> (seconds since 1Jan1904=w1762:timestamp)
                n915 = To Double Precision Float(number=w1762) -> (double precision float=w1761:dbl)
                n916 = local write "Time Stamp (s)"(w1761) -> ()
              }
            }
            n917 = property on="Z-Stack Measure" class="Bool (strict)"(error in=w1753, "Val(Sgnl)"=TRUE ("Value (Signaling)")) -> (error out=w1752:errorcluster)  [unwired: 1 in, 1 out]
          }
          frame True {
            w1774 = FALSE ("2D Time-Lapse Measure")
            n918 = local write "Current 3D Time-Lapse Meas"(0 ("Current Slice")) -> ()
            n919 = local write "3D Time-Lapse Measure"(w1774) -> ()
            n920 = local write "Stop 3D Time-Lapse"(w1774) -> ()
          }
        }
      }
      event "Lifetime Selection", "Min Lifetime (s)", "Max Lifetime (s)", "Bins", "Max Intensity", "Min Intensity", "Auto Scale?": Value Change {
        w1791 = 100.0 ("y")
        n921 = event-data() -> ()  [unwired: 1 in, 1 out]
        n922 = local read "Lifetime Selection"() -> (w1817:enum32{"1w Lifetime", "DC&1w Lifetime"})
        n923 = case shown="\"DC&1w Lifetime\"" w1817 {
          tunnel: [w1819 w1820] -> w1812
          frame "1w Lifetime", Default {
            n924 = local read "1w Lifetime (s)"() -> (w1819:dbl[][])
          }
          frame "DC&1w Lifetime" {
            n925 = local read "DC&1w Lifetime (s)"() -> (w1820:dbl[][])
          }
        }
        n926 = local read "Auto Scale?"() -> (w1809:bool)
        n927 = local read "Max Lifetime (s)"() -> (w1786:dbl)
        n928 = local read "Max Intensity"() -> (w1811:dbl)
        n929 = local read "Min Lifetime (s)"() -> (w1785:dbl)
        n930 = local read "Min Intensity"() -> (w1810:dbl)
        n931 = local read "V_DC"() -> (w1801:dbl[][])
        n932 = call "HSVCombIntensityLifetime.vi"("min_intensity"=w1810, "Auto Scale?"=w1809, "max_intensity"=w1811, "lifetime_max (s)"=w1786, "lifetime_min (s)"=w1785, "Lifetime image"=w1812, "Intensity image"=w1801) -> ("Min"=w1778:dbl, "Max"=w1779:dbl, "Lifetime Color Ramp"=w1816:i32[][], "HSV to RGB Picture"=w1815:picture)  [unwired: 1 in]
        n933 = Array Max & Min(array=w1801) -> (max value=w1800:dbl, min value=w1798:dbl)  [unwired: 2 out]
        n934 = local write "Lifetime Color Ramp"(w1816) -> ()
        n935 = local write "Composite Image"(w1815) -> ()
        n936 = Subtract(x=w1778, y=w1798) -> (x-y=w1797:dbl)
        n937 = Subtract(x=w1800, y=w1798) -> (x-y=w1796:dbl)
        n938 = Subtract(x=w1779, y=w1798) -> (x-y=w1799:dbl)
        n939 = control-ref of="V_DC"() -> (w1780:refnum<vi>)
        n940 = Divide(x=w1799, y=w1796) -> (x/y=w1795:dbl)
        n941 = Divide(x=w1797, y=w1796) -> (x/y=w1793:dbl)
        n942 = Multiply(x=w1795, y=w1791) -> (x*y=w1794:dbl)
        n943 = Multiply(x=w1793, y=w1791) -> (x*y=w1792:dbl)
        n944 = local write "Max Intensity"(w1779) -> ()
        n945 = local write "Min Intensity"(w1778) -> ()
        n946 = local write "Max (%)"(w1794) -> ()
        n947 = property class="IntGraph (strict)"(reference=w1780, error in=w1782, "ZScale.Maximum"=w1779, "ZScale.Minimum"=w1778) -> (error out=w1781:errorcluster)  [unwired: 1 out]
        n948 = local write "Min (%)"(w1792) -> ()
        n949 = local read "Measurement Parameters"() -> (w1814:T4)
        n950 = local read "Bins"() -> (w1804:i32)
        n951 = local read "1w Lifetime (s)"() -> (w1808:dbl[][])
        n952 = local read "DC&1w Lifetime (s)"() -> (w1807:dbl[][])
        n953 = Unbundle By Name(w1814) -> ("Pixel Size"=w1813:dbl)
        n954 = control-ref of="1w Lifetime Hist"() -> (w1806:refnum<vi>)
        n955 = control-ref of="DC&1w Lifetime Hist"() -> (w1805:refnum<vi>)
        n956 = control-ref of="Lifetime Color Ramp"() -> (w1788:refnum<vi>)
        n957 = control-ref of="Composite Image"() -> (w1789:refnum<vi>)
        n958 = To Long Integer(number=w1813) -> (32bit integer=w1787:i32)
        n959 = Square(x=w1787) -> (x^2=w1790:i32)
        n960 = call "LifetimeHistogram.vi"("1w Lifetime"=w1808, "DC&1w Lifetime"=w1807, "1w reference"=w1806, "DC&1w reference"=w1805, "Data Size"=w1790, "error in (no error)"=w1781, "Bins"=w1804) -> ("error out"=w1783:errorcluster, "1w Lifetime Hist"=w1803:T7, "DC&1w Lifetime Hist"=w1802:T7)  [unwired: 6 in, 4 out]
        n961 = call "CompositeProperties.vi"("Image Reference"=w1789, "Ramp Reference"=w1788, "Pixel Size"=w1787, "Max Lifetime (s)"=w1786, "Min Lifetime (s)"=w1785, "error in (no error)"=w1783) -> ("error out"=w1784:errorcluster)  [unwired: 13 in]
        n962 = local write "1w Lifetime Hist"(w1803) -> ()
        n963 = local write "DC&1w Lifetime Hist"(w1802) -> ()
      }
      event "Max (%)", "Min (%)": Value Change {
        w1829 = 100.0 ("y")
        w1854 = 100.0 ("y")
        n964 = event-data() -> ()  [unwired: 1 in, 1 out]
        n965 = local read "V_DC"() -> (w1858:dbl[][])
        n966 = Array Max & Min(array=w1858) -> (max value=w1857:dbl, min value=w1848:dbl)  [unwired: 2 out]
        n967 = Divide(x="Max (%)", y=w1854) -> (x/y=w1853:dbl)
        n968 = Divide(x="Min (%)", y=w1854) -> (x/y=w1852:dbl)
        n969 = Subtract(x=w1857, y=w1848) -> (x-y=w1851:dbl)
        n970 = Multiply(x=w1853, y=w1851) -> (x*y=w1850:dbl)
        n971 = Multiply(x=w1852, y=w1851) -> (x*y=w1849:dbl)
        n972 = Add(x=w1850, y=w1848) -> (x+y=w1840:dbl)
        n973 = Add(x=w1849, y=w1848) -> (x+y=w1839:dbl)
        n974 = local read "Lifetime Selection"() -> (w1847:enum32{"1w Lifetime", "DC&1w Lifetime"})
        n975 = case shown="\"DC&1w Lifetime\"" w1847 {
          tunnel: [w1860 w1861] -> w1844
          frame "1w Lifetime", Default {
            n976 = local read "1w Lifetime (s)"() -> (w1860:dbl[][])
          }
          frame "DC&1w Lifetime" {
            n977 = local read "DC&1w Lifetime (s)"() -> (w1861:dbl[][])
          }
        }
        n978 = local read "Auto Scale?"() -> (w1843:bool)
        n979 = local read "Max Lifetime (s)"() -> (w1842:dbl)
        n980 = local read "V_DC"() -> (w1828:dbl[][])
        n981 = local read "Min Lifetime (s)"() -> (w1841:dbl)
        n982 = call "HSVCombIntensityLifetime.vi"("min_intensity"=w1839, "Auto Scale?"=w1843, "max_intensity"=w1840, "lifetime_max (s)"=w1842, "lifetime_min (s)"=w1841, "Lifetime image"=w1844, "Intensity image"=w1828) -> ("Min"=w1823:dbl, "Max"=w1824:dbl, "Lifetime Color Ramp"=w1846:i32[][], "HSV to RGB Picture"=w1845:picture)  [unwired: 1 in]
        n983 = Array Max & Min(array=w1828) -> (max value=w1838:dbl, min value=w1836:dbl)  [unwired: 2 out]
        n984 = Subtract(x=w1823, y=w1836) -> (x-y=w1835:dbl)
        n985 = Subtract(x=w1838, y=w1836) -> (x-y=w1834:dbl)
        n986 = Subtract(x=w1824, y=w1836) -> (x-y=w1837:dbl)
        n987 = local write "Lifetime Color Ramp"(w1846) -> ()
        n988 = local write "Composite Image"(w1845) -> ()
        n989 = Divide(x=w1837, y=w1834) -> (x/y=w1833:dbl)
        n990 = Divide(x=w1835, y=w1834) -> (x/y=w1831:dbl)
        n991 = control-ref of="V_DC"() -> (w1827:refnum<vi>)
        n992 = Multiply(x=w1833, y=w1829) -> (x*y=w1832:dbl)
        n993 = Multiply(x=w1831, y=w1829) -> (x*y=w1830:dbl)
        n994 = local write "Max (%)"(w1832) -> ()
        n995 = local write "Min (%)"(w1830) -> ()
        n996 = local write "Max Intensity"(w1824) -> ()
        n997 = local write "Min Intensity"(w1823) -> ()
        n998 = property class="IntGraph (strict)"(reference=w1827, error in=w1826, "ZScale.Maximum"=w1824, "ZScale.Minimum"=w1823) -> (error out=w1825:errorcluster)  [unwired: 1 out]
      }
      event "Phasor Plot": Mouse Move; "Phasor Plot": Mouse Down {
        n999 = event-data() -> ("Coords.Horizontal"=w1899:i32, "Coords.Vertical"=w1898:i32, "Type"=w1893:T17)  [unwired: 1 in]
        n1000 = control-ref of="Phasor Plot"() -> (w1900:refnum<vi>)
        n1001 = property on="Property Node" class="IntGraph (strict)"(reference=w1900, error in=w1918, "Width"="PicSize", "Height"="PicSize") -> (error out=w1888:errorcluster, "XScale.Maximum"=w1917:dbl, "XScale.Minimum"=w1911:dbl, "YScale.Maximum"=w1906:dbl, "YScale.Minimum"=w1907:dbl, "Plot Bounds"=w1910:T18)  [unwired: 1 out]
        n1002 = Unbundle By Name(w1910) -> ("Left"=w1916:i16, "Top"=w1909:i16)
        n1003 = Subtract(x=w1899, y=w1916) -> (x-y=w1895:i32)
        n1004 = Subtract(x=w1898, y=w1909) -> (x-y=w1894:i32)
        n1005 = Subtract(x=w1917, y=w1911) -> (x-y=w1915:dbl)
        n1006 = Subtract(x=w1906, y=w1907) -> (x-y=w1914:dbl)
        n1007 = Divide(x=w1915, y="PicSize") -> (x/y=w1913:dbl)
        n1008 = Divide(x=w1914, y="PicSize") -> (x/y=w1908:dbl)
        n1009 = Multiply(x=w1895, y=w1913) -> (x*y=w1912:dbl)
        n1010 = Multiply(x=w1894, y=w1908) -> (x*y=w1905:dbl)
        n1011 = local read "LaserRepRate (Hz)"() -> (w1862:dbl)
        n1012 = Add(x=w1912, y=w1911) -> (x+y=w1884:dbl)
        "G" <- w1884
        n1013 = Subtract(x=w1906, y=w1905) -> (x-y=w1883:dbl)
        "S" <- w1883
        n1014 = Bundle(w1884, w1883) -> (w1896:cluster{dbl, dbl})  [unwired: 1 in]
        n1015 = Multiply(x=w1862, y=6.283185307179586) -> (x*y=w1902:dbl)
        n1016 = Divide(x=w1883, y=w1884) -> (x/y=w1903:dbl)
        n1017 = Divide(x=w1903, y=w1902) -> (x/y=→"[tau]":dbl)
        n1018 = case shown="\"ROI1\", Default" "ROI Select" {
          tunnel: [w1919 w1920 w1921 w1922] -> w1890
          frame "ROI1", Default {
            n1019 = local read "Center1"() -> (w1919:cluster{dbl, dbl})
          }
          frame "ROI2" {
            n1020 = local read "Center2"() -> (w1920:cluster{dbl, dbl})
          }
          frame "ROI3" {
            n1021 = local read "Center3"() -> (w1921:cluster{dbl, dbl})
          }
          frame "ROI4" {
            n1022 = local read "Center4"() -> (w1922:cluster{dbl, dbl})
          }
        }
        n1023 = property on="Phasor Plot" class="IntGraph (strict)"(error in=w1888) -> (error out=w1887:errorcluster, "PlotImages.Front"=w1886:picture)  [unwired: 1 in, 1 out]
        n1024 = local read "Radius4"() -> (w1871:dbl)
        n1025 = local read "Center4"() -> (w1870:cluster{dbl, dbl})
        n1026 = local read "Radius2"() -> (w1875:dbl)
        n1027 = local read "Center2"() -> (w1874:cluster{dbl, dbl})
        n1028 = local read "Radius3"() -> (w1873:dbl)
        n1029 = local read "Center3"() -> (w1872:cluster{dbl, dbl})
        n1030 = local read "Radius1"() -> (w1877:dbl)
        n1031 = local read "Center1"() -> (w1876:cluster{dbl, dbl})
        n1032 = local read "PicSize"() -> (w1869:u32)
        n1033 = case shown="\"Mouse Move\", Default" w1893 {
          tunnel: w1896 -> [w1925 w1962]
          tunnel: [w1927 w1963] -> w1892
          tunnel: w1887 -> [w1928 w1964]
          tunnel: [w1928 w1964] -> w1891
          tunnel: w1890 -> [_ w1961]
          tunnel: w1886 -> [w1927 w1959]
          tunnel: "ROI Select" -> [w1926 w1958]
          tunnel: w1877 -> [_ w1957]
          tunnel: w1876 -> [_ w1956]
          tunnel: "Color1" -> [_ w1955]
          tunnel: w1875 -> [_ w1954]
          tunnel: w1874 -> [_ w1953]
          tunnel: "Color2" -> [_ w1952]
          tunnel: w1873 -> [_ w1951]
          tunnel: w1872 -> [_ w1950]
          tunnel: "Color3" -> [_ w1949]
          tunnel: w1871 -> [_ w1948]
          tunnel: w1870 -> [_ w1947]
          tunnel: "Color4" -> [_ w1946]
          tunnel: "ROI4?" -> [_ w1945]
          tunnel: "ROI2?" -> [_ w1944]
          tunnel: "ROI1?" -> [_ w1943]
          tunnel: w1869 -> [_ w1942]
          tunnel: "ROI3?" -> [_ w1941]
          frame "Mouse Down" {
            w1923 = TRUE ("ROI Drawing")
            n1034 = case shown="\"ROI4\"" w1926 {
              tunnel: w1925 -> [_ w1931 w1934 w1937 w1940]
              tunnel: 0.0 ("Radius2") -> [_ w1930 w1933 w1936 w1939]
              tunnel: w1923 -> [_ w1929 w1932 w1935 w1938]
              frame "None" {
              }
              frame "ROI1" {
                n1035 = local write "Radius1"(w1930) -> ()
                n1036 = local write "ROI1?"(w1929) -> ()
                "Center1" <- w1931
              }
              frame "ROI2" {
                n1037 = local write "Radius2"(w1933) -> ()
                n1038 = local write "ROI2?"(w1932) -> ()
                "Center2" <- w1934
              }
              frame "ROI3" {
                n1039 = local write "Radius3"(w1936) -> ()
                n1040 = local write "ROI3?"(w1935) -> ()
                "Center3" <- w1937
              }
              frame "ROI4" {
                n1041 = local write "Radius4"(w1939) -> ()
                n1042 = local write "ROI4?"(w1938) -> ()
                "Center4" <- w1940
              }
            }
            "ROI Drawing" <- w1923
          }
          frame "Mouse Move", Default {
            n1043 = local read "ROI Drawing"() -> (w1960:bool)
            n1044 = case shown="True" w1960 {
              tunnel: [w1965 w1987] -> w1963
              tunnel: w1962 -> [_ w2001]
              tunnel: w1961 -> [_ w2000]
              tunnel: w1959 -> [w1965 _]
              tunnel: w1958 -> [_ w1992]
              tunnel: w1957 -> [_ w1985]
              tunnel: w1956 -> [_ w1984]
              tunnel: w1955 -> [_ w1983]
              tunnel: w1954 -> [_ w1982]
              tunnel: w1953 -> [_ w1972]
              tunnel: w1952 -> [_ w1980]
              tunnel: w1951 -> [_ w1979]
              tunnel: w1950 -> [_ w1971]
              tunnel: w1949 -> [_ w1978]
              tunnel: w1948 -> [_ w1975]
              tunnel: w1947 -> [_ w1974]
              tunnel: w1946 -> [_ w1973]
              tunnel: w1945 -> [_ w1976]
              tunnel: w1944 -> [_ w1981]
              tunnel: w1943 -> [_ w1986]
              tunnel: w1942 -> [_ w1990]
              tunnel: w1941 -> [_ w1966]
              frame False {
              }
              frame True {
                n1045 = Subtract(x=w2000, y=w2001) -> (x-y=w1999:cluster{dbl, dbl})
                n1046 = call "Empty Picture"() -> ("empty picture"=w1991:picture)
                n1047 = Unbundle(w1999) -> (w1998:dbl, w1997:dbl)
                n1048 = local read "G_max"() -> (w1970:dbl)
                n1049 = local read "G_min"() -> (w1969:dbl)
                n1050 = local read "S_max"() -> (w1968:dbl)
                n1051 = local read "S_min"() -> (w1967:dbl)
                n1052 = Square(x=w1998) -> (x^2=w1996:dbl)
                n1053 = Square(x=w1997) -> (x^2=w1995:dbl)
                n1054 = Add(x=w1996, y=w1995) -> (x+y=w1994:dbl)
                n1055 = Square Root(x=w1994) -> (sqrt(x)=w1993:dbl)
                n1056 = call "DrawROICircle.vi"("old picture"=w1991, "ROI?"=w1986, "Radius (G/S)"=w1985, "Center (G/S)"=w1984, "PicSize"=w1990, "Color"=w1983, "G_max"=w1970, "S_max"=w1968, "G_min"=w1969, "S_min"=w1967) -> ("new picture"=w1989:picture)  [unwired: 9 in]
                n1057 = call "DrawROICircle.vi"("old picture"=w1989, "ROI?"=w1981, "Radius (G/S)"=w1982, "Center (G/S)"=w1972, "PicSize"=w1990, "Color"=w1980, "G_max"=w1970, "S_max"=w1968, "G_min"=w1969, "S_min"=w1967) -> ("new picture"=w1977:picture)  [unwired: 9 in]
                n1058 = call "DrawROICircle.vi"("old picture"=w1977, "ROI?"=w1966, "Radius (G/S)"=w1979, "Center (G/S)"=w1971, "PicSize"=w1990, "Color"=w1978, "G_max"=w1970, "S_max"=w1968, "G_min"=w1969, "S_min"=w1967) -> ("new picture"=w1988:picture)  [unwired: 9 in]